vi "Main.vi"() -> ()   [LabVIEW 2020] (continued)
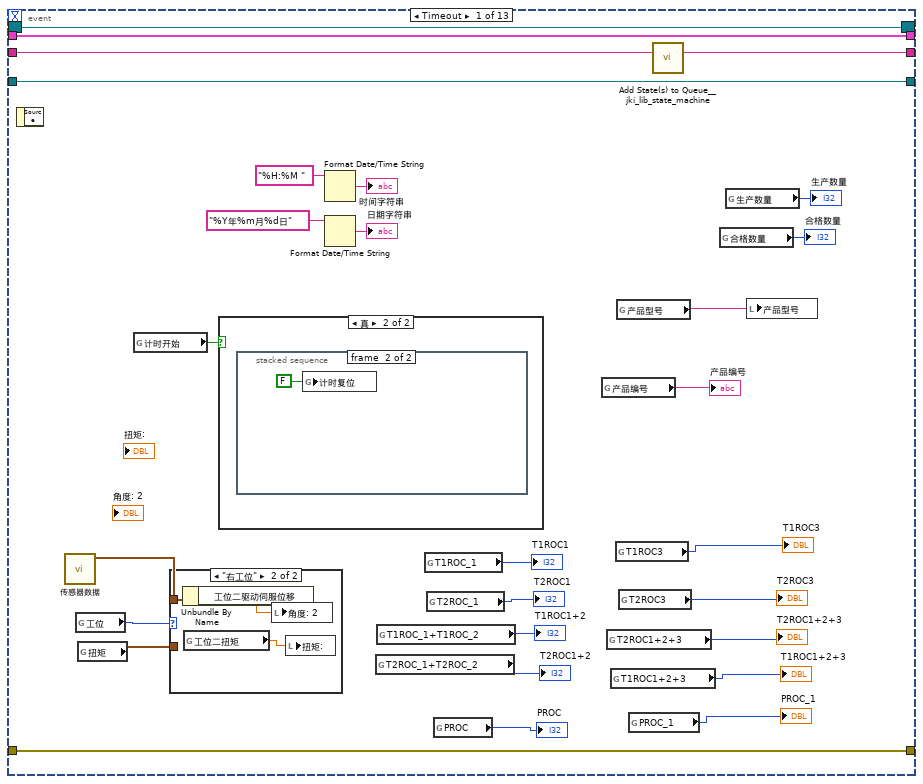
[diagram p2: hidden frame]
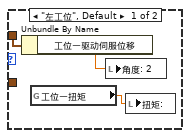
[diagram p3: hidden frame]
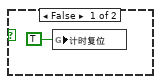
[diagram p4: hidden frame]
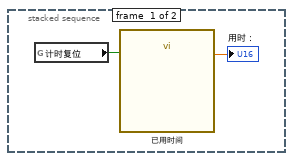
[diagram p5: hidden frame]
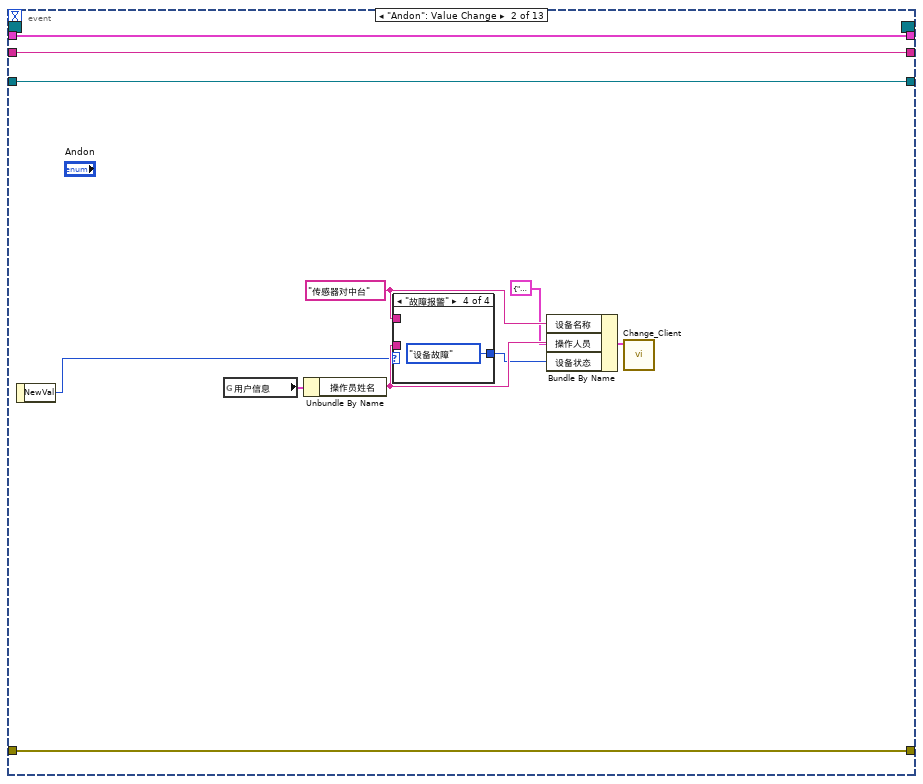
[diagram p6: hidden frame]
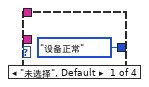
[diagram p7: hidden frame]
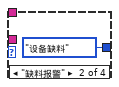
[diagram p8: hidden frame]
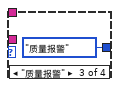
[diagram p9: hidden frame]
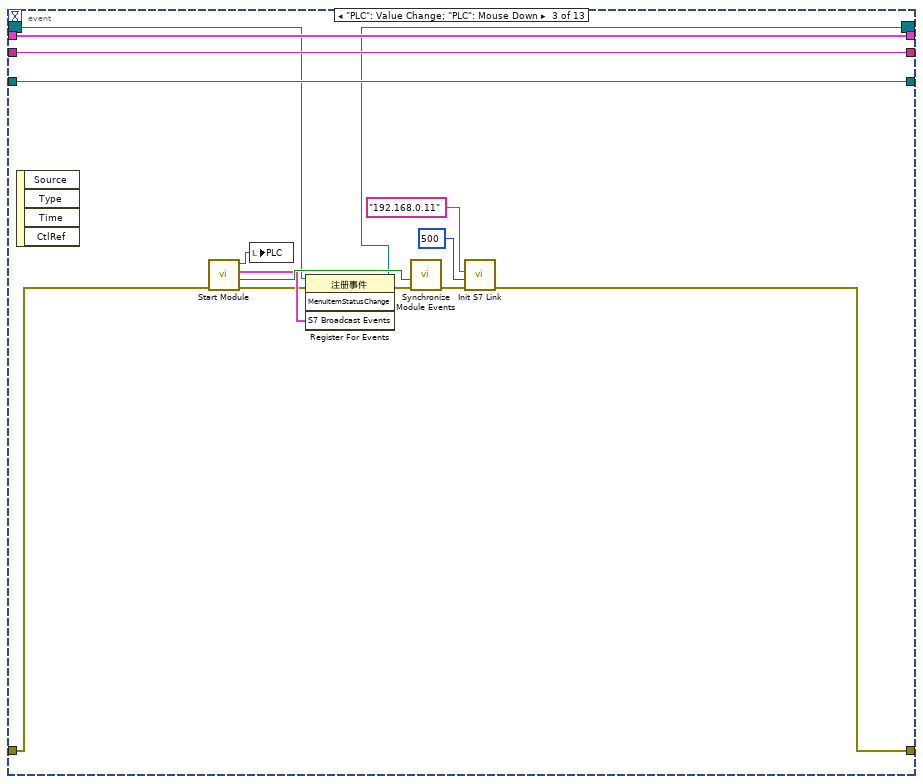
[diagram p10: hidden frame]
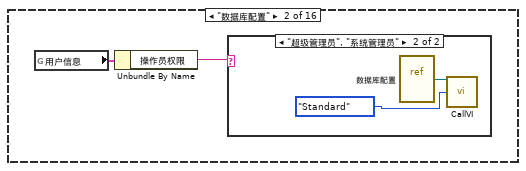
[diagram p12: hidden frame]
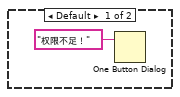
[diagram p13: hidden frame]
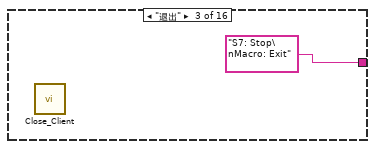
[diagram p14: hidden frame]
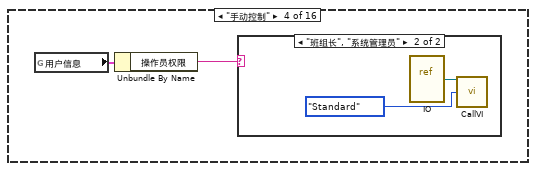
[diagram p15: hidden frame]
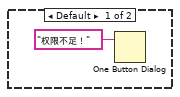
[diagram p16: hidden frame]
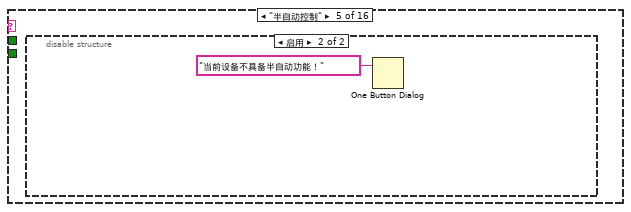
[diagram p17: hidden frame]
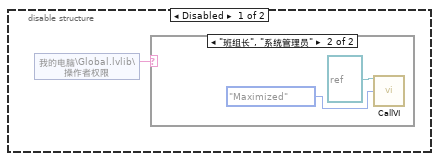
[diagram p18: hidden frame]
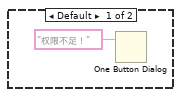
[diagram p19: hidden frame]
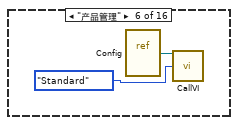
[diagram p20: hidden frame]
            }
            n123 = call <vilib>:"Add State(s) to Queue__jki_lib_state_machine.vi"("State(s) in (\"\")"=w114, "State(s) at Back (\"\")"=w107) -> ("States Out"=w112:string)  [unwired: 13 in]
          }
          event User Event {
            n124 = event-data() -> ("Init?"=w181:bool)  [unwired: 1 in, 1 out]
            n125 = local write "PLC"(w181) -> ()
            n126 = call <vilib>:"Add State(s) to Queue__jki_lib_state_machine.vi"("State(s) in (\"\")"=w176) -> ("States Out"=w177:string)  [unwired: 14 in]
          }
          event User Event {
            n127 = event-data() -> ("Running?"=w188:bool)  [unwired: 1 in]
            n128 = local write "PLC"(w188) -> ()
            n129 = call <vilib>:"Add State(s) to Queue__jki_lib_state_machine.vi"("State(s) in (\"\")"=w183) -> ("States Out"=w184:string)  [unwired: 14 in]
          }
          event User Event {
            n130 = event-data() -> ()  [unwired: 1 in, 7 out]
            n131 = local write "PLC"(FALSE ("PLC")) -> ()
            n132 = call <vilib>:"Add State(s) to Queue__jki_lib_state_machine.vi"("State(s) in (\"\")"=w192) -> ("States Out"=w193:string)  [unwired: 14 in]
          }
          event User Event {
            n133 = event-data() -> ("Error"=w204:errorcluster)  [unwired: 1 in]
            n134 = Merge Errors(w204, w203) -> (w202:errorcluster)
            n135 = disable-structure shown="禁用" {
              disable-tunnel: ["S7: Stop\nS7: Initialize\nIdle" _] -> w197
              frame Disabled {
              }
              frame Enabled {
              }
            }
            n136 = call <vilib>:"Add State(s) to Queue__jki_lib_state_machine.vi"("State(s) in Front (\"\")"=w197, "State(s) in (\"\")"=w199) -> ("States Out"=w200:string)  [unwired: 13 in]
          }
          event "自动": Mouse Down {
            n137 = event-data() -> ()  [unwired: 1 in, 1 out]
            n138 = local read "自动"() -> (w206:bool)
            n139 = case shown="假" w206 {
              frame False {
                n140 = global read "Global.vi" "工位"() -> (w213:enum16{"左工位", "右工位"})
                n141 = case shown="\"左工位\", 默认" w213 {
                  frame "左工位", Default {
                    n142 = call "设备状态.vi"("工位"=enum16{"工位一", "工位二"}."工位一") -> ("Status_Read"=w215:i16)  [unwired: 10 in]
                    n143 = case shown="5" w215 {
                      frame 0, Default {
                        n144 = One Button Dialog(message="请复位！" ("消息")) -> ()  [unwired: 1 in, 1 out]
                        n145 = call "设备状态.vi"("枚举"=enum16{"Read", "Write"}."Write", "工位"=enum16{"工位一", "工位二"}."工位一", "Status_Write"=i16 0) -> ()  [unwired: 8 in, 1 out]
                      }
                      frame 5 {
                        n146 = vi-ref "Auto.vi"() -> (w222:refnum<vi>)
                        n147 = invoke class="VI" method="Ctrl Val.Set"(reference=w222, "Control Name"="STEP" ("控件名"), "Value"="进入自动" ("控件名")) -> ()  [unwired: 2 in, 5 out]
                      }
                    }
                  }
                  frame "右工位" {
                    n148 = call "设备状态.vi"("工位"=enum16{"工位一", "工位二"}."工位二") -> ("Status_Read"=w224:i16)  [unwired: 10 in]
                    n149 = case shown="5" w224 {
                      frame 0, Default {
                        n150 = One Button Dialog(message="请复位！" ("消息")) -> ()  [unwired: 1 in, 1 out]
                        n151 = call "设备状态.vi"("枚举"=enum16{"Read", "Write"}."Write", "工位"=enum16{"工位一", "工位二"}."工位二", "Status_Write"=i16 0) -> ()  [unwired: 8 in, 1 out]
                      }
                      frame 5 {
                        n152 = vi-ref "Auto2.vi"() -> (w231:refnum<vi>)
                        n153 = invoke class="VI" method="Ctrl Val.Set"(reference=w231, "Control Name"="STEP" ("控件名"), "Value"="进入自动" ("控件名")) -> ()  [unwired: 2 in, 5 out]
                      }
                    }
                  }
                }
              }
              frame True {
                n154 = global read "Global.vi" "工位"() -> (w232:enum16{"左工位", "右工位"})
                n155 = case shown="\"左工位\", 默认" w232 {
                  frame "左工位", Default {
                    n156 = Two Button Dialog(message="确定要退出自动？" ("消息")) -> (T button?=w233:bool)  [unwired: 2 in]
                    n157 = case shown="真" w233 {
                      frame False {
                      }
                      frame True {
                        n158 = vi-ref "Auto.vi"() -> (w237:refnum<vi>)
                        n159 = invoke class="VI" method="Ctrl Val.Set"(reference=w237, "Control Name"="STEP" ("控件名"), "Value"="退出自动" ("控件名")) -> ()  [unwired: 2 in, 5 out]
                      }
                    }
                  }
                  frame "右工位" {
                    n160 = Two Button Dialog(message="确定要退出自动？" ("消息")) -> ()  [unwired: 2 in, 1 out]
                    n161 = vi-ref "Auto2.vi"() -> (w240:refnum<vi>)
                    n162 = invoke class="VI" method="Ctrl Val.Set"(reference=w240, "Control Name"="STEP" ("控件名"), "Value"="退出自动" ("控件名")) -> ()  [unwired: 2 in, 5 out]
                  }
                }
              }
            }
            n163 = call <vilib>:"Add State(s) to Queue__jki_lib_state_machine.vi"("State(s) in (\"\")"=w209) -> ("States Out"=w210:string)  [unwired: 14 in]
          }
          event "布尔": Mouse Down {
            n164 = event-data() -> ()  [unwired: 1 in, 8 out]
            n165 = vi-ref "System.vi"() -> (w249:refnum<vi>)
            n166 = call "CallVI.vi"("VI引用"=w249, "状态"=T4."Standard") -> ()  [unwired: 12 in, 2 out]
            n167 = call <vilib>:"Add State(s) to Queue__jki_lib_state_machine.vi"("State(s) in (\"\")"=w245) -> ("States Out"=w244:string)  [unwired: 14 in]
          }
          event "错误": Mouse Down {
            n168 = event-data() -> ()  [unwired: 1 in, 8 out]
            n169 = vi-ref "报警信息.vi"() -> (w252:refnum<vi>)
            n170 = call "CallVI.vi"("VI引用"=w252, "状态"=T4."Standard") -> ()  [unwired: 12 in, 2 out]
            n171 = call <vilib>:"Add State(s) to Queue__jki_lib_state_machine.vi"("State(s) in (\"\")"=w254) -> ("States Out"=w255:string)  [unwired: 14 in]
          }
          event Panel Close? {
            n172 = event-data() -> ()  [unwired: 1 in, 1 out]
            n173 = global write "Global.vi" "程序关闭"(TRUE ("程序关闭")) -> ()
            n174 = call <vilib>:"Add State(s) to Queue__jki_lib_state_machine.vi"("State(s) in Front (\"\")"="S7: Stop\nMacro: Exit", "State(s) in (\"\")"=w264) -> ("States Out"=w263:string)  [unwired: 13 in]
            n175 = event-data("Discard?"=TRUE) -> ()  [unwired: 1 in, 1 out]
          }
          event "更换产品": Value Change {
            n176 = event-data() -> ("NewVal"=w266:refnum<vi>)  [unwired: 1 in, 5 out]
            n177 = stacked-sequence {
              tunnel: w266 -> [w271]
              frame #0 {
                n178 = stacked-sequence {
                  tunnel: w271 -> [w272]
                  frame #0 {
                    n179 = disable-structure shown="禁用" {
                      disable-tunnel: w272 -> [w274 _]
                      frame Disabled {
                        n180 = call "Call_SubPanal.vi"("VI引用句柄"=w274) -> ("SubPnl引用句柄"=w273:refnum<vi>)  [unwired: 9 in, 1 out]
                      }
                      frame Enabled {
                      }
                    }
                  }
                }
              }
            }
            n181 = call <vilib>:"Add State(s) to Queue__jki_lib_state_machine.vi"("State(s) in (\"\")"=w267) -> ("States Out"=w268:string)  [unwired: 14 in]
          }
        }
      }
      frame "---------- Core ----------" {
        n182 = call <vilib>:"Add State(s) to Queue__jki_lib_state_machine.vi"("State(s) in (\"\")"=w280) -> ("States Out"=w279:string)  [unwired: 14 in]
      }
      frame Default {
        w292 = 42 items=["No error", "Argument error", "Memory is full", "Out of zone", "End of file", "File already open", "Generic file I/O error", "File not found", "File permission error", "Disk is full", "Duplicate path", "Too many files open", "System feature not enabled", "Resource file not found", "Cannot add resource", "Resource not found", "Image not found", "Image memory error", "Pen does not exist", "Config type invalid", "Config token not found", "Config parse error", "Config memory error", "Bad external code format", "Bad external code offset", "External code not present", "Null window", "Destroy window error", "Null menu", "Print aborted", "Bad print record", "Print driver error", "Windows error during printing", "Memory error during printing", "Print dialog error", "Generic print error", "Invalid device refnum", "Device not found", "Device parameter error", "Device unit error", "Cannot open device", "Device call aborted", "Generic error", "Cancelled by user", "Object ID too low", "Object ID too high", "Object not in heap", "Unknown heap", "Unknown object (invalid DefProc)", "Unknown object (DefProc not in table)", "Message out of range", "Invalid (null) method", "Unknown message", "Manager call not supported", "Bad address", "Network operation in progress", "Network operation timed out", "Connection is busy", "Network attribute not supported", "Network error", "Address in use", "System out of memory", "Connection aborted", "Connection refused", "Not connected", "Already connected", "Connection closed", "Initialization error (interapplication manager)", "Bad occurrence", "Wait on unbound occurrence handler", "Occurrence queue overflow", "Datalog type conflict", "Unused", "Unrecognized type (interapplication manager)", "Memory corrupt", "Failed to make temporary DLL", "Old CIN version", "Drag socket not found", "Failed to load drop-object", "Failed to register OLE object", "Failed to release OLE object", "Format specifier type mismatch", "Unknown format specifier", "Too few format specifiers", "Too many format specifiers", "Scan failed", "Newer CIN version", "Error converting to variant", "Runtime menu error", "Password tampered", "Variant attribute not found", "Incompatible variant data type", "Event data is not available", "Event Store is not present", "Occurrence is not found", "Event Queue is not created", "Event info is not available", "Refnum passed is NULL", "Error retrieving Class GUID", "Error retrieving CoClass GUID", "Error retrieving TypeLib GUID.", "Bad built application magic bytes.", "Specific driver is different from the specific driver associated with the Logical Name.", "There is no session opened to the class driver.", "Max Error", "MAX - Error with config objects", "MAX - Error loading configuration", "MAX - Group not supported"]
        # "Current State"
        n183 = Format Into String(format string="Software Exception: Unhandled State \"%s\"." ("message"), error in=w288, w283) -> (resulting string=w291:string, error out=w290:errorcluster)  [unwired: 1 in]
        n184 = call <vilib>:"Error Cluster From Error Code.vi"("show call chain? (False)"=TRUE, "error in (no error)"=w290, "error message (\"\")"=w291, "error code (0)"=w292) -> ("error out"=w289:errorcluster)  [unwired: 5 in]
        n185 = call <vilib>:"Add State(s) to Queue__jki_lib_state_machine.vi"("State(s) in (\"\")"=w287) -> ("States Out"=w286:string)  [unwired: 14 in]
      }
      frame "Initialize Core Data" {
        # "originally closed?"
        # "exe?"
        n186 = property class="VI"() -> ("Front Panel.Open"=w303:bool)  [unwired: 2 in, 2 out]
        n187 = property class="App"() -> ("App.Kind"=w302:T5)  [unwired: 2 in, 2 out]
        n188 = control-ref of="Current VI Reference"() -> (w296:refnum<vi>)
        n189 = Not(x=w303) -> (.not. x?=w300:bool)
        n190 = Equal?(x=w302, y=T5."Run Time System" ("Application:Kind")) -> (x = y?=w299:bool)
        n191 = Or(x=w300, y=w299) -> (x .or. y?=w297:bool)
        n192 = Bundle By Name(cluster=w298, "Core.Current VI Reference"=w296, "Core.Close Panel on Exit?"=w297) -> (w305:T8)
        n193 = call <vilib>:"Add State(s) to Queue__jki_lib_state_machine.vi"("State(s) in (\"\")"=w307) -> ("States Out"=w306:string)  [unwired: 14 in]
      }
      frame "Error Handler" {
        n194 = call <vilib>:"General Error Handler.vi"("error in (no error)"=w311) -> ()  [unwired: 10 in, 5 out]
        n195 = call <vilib>:"Add State(s) to Queue__jki_lib_state_machine.vi"("State(s) in Front (\"\")"="/* Post Error States", "State(s) in (\"\")"=w315) -> ("States Out"=w314:string)  [unwired: 13 in]
      }
      frame "Exit" {
        n196 = call <vilib>:"Add State(s) to Queue__jki_lib_state_machine.vi"("State(s) in (\"\")"=w322) -> ("States Out"=w321:string)  [unwired: 14 in]
      }
      frame "--------- Library --------" {
        n197 = call <vilib>:"Add State(s) to Queue__jki_lib_state_machine.vi"("State(s) in (\"\")"=w328) -> ("States Out"=w327:string)  [unwired: 14 in]
      }
      frame "S7: Initialize" {
        n198 = property on="PLC" class="Bool (严格)"("Val(Sgnl)"=FALSE ("值(信号)")) -> ()  [unwired: 2 in, 2 out]
      }
      frame "S7: Stop" {
        n199 = call "Stop Module.vi"("error in (no error)"=w337) -> ("error out"=w336:errorcluster)  [unwired: 10 in]
        n200 = call <vilib>:"Add State(s) to Queue__jki_lib_state_machine.vi"("State(s) in (\"\")"=w338) -> ("States Out"=w339:string)  [unwired: 14 in]
      }
      frame "---------- Data ----------" {
        n201 = call <vilib>:"Add State(s) to Queue__jki_lib_state_machine.vi"("State(s) in (\"\")"=w347) -> ("States Out"=w346:string)  [unwired: 14 in]
      }
      frame "Data: Initialize" {
        w353 = T9 {"Current VI Reference"=refnum, "Close Panel on Exit?"=FALSE}  # Core
        w355 = TRUE  # Your Boolean data
        w354 = ""  # Your string data
        n202 = vi-ref "扭矩.vi"() -> (w349:refnum<vi>)
        n203 = call "CallVI.vi"("VI引用"=w349, "状态"=T4."Hidden") -> ()  [unwired: 12 in, 2 out]
        n204 = global write "Global.vi" "计时开始"(FALSE ("计时结束")) -> ()
        n205 = Bundle("Core"=w353, "Your Boolean data"=w355, "Your string data"=w354) -> (w357:T8)  [unwired: 1 in]
        n206 = call <vilib>:"Add State(s) to Queue__jki_lib_state_machine.vi"("State(s) in (\"\")"=w359) -> ("States Out"=w358:string)  [unwired: 14 in]
      }
      frame "Data: Cleanup" {
        n207 = Unbundle By Name(w362) -> ("Core.Current VI Reference"=w365:refnum<vi>)
        n208 = Close Reference(reference=w365, error in (no error)=w364) -> (error out=w363:errorcluster)
        n209 = call <vilib>:"Add State(s) to Queue__jki_lib_state_machine.vi"("State(s) in (\"\")"=w367) -> ("States Out"=w366:string)  [unwired: 14 in]
      }
      frame "---------- UI ----------" {
        # "Do not put any code in this frame.\n(It is a separator no-op. You can make a copy of this frame to create a new UI frame)"
        n210 = call <vilib>:"Add State(s) to Queue__jki_lib_state_machine.vi"("State(s) in (\"\")"=w373) -> ("States Out"=w372:string)  [unwired: 14 in]
      }
      frame "UI: Initialize" {
        n211 = global read "Global.vi" "工位"() -> (w374:enum16{"左工位", "右工位"})
        n212 = disable-structure shown="禁用" {
          frame Disabled {
            n213 = vi-ref "Auto2.vi"() -> (w396:refnum<vi>)
            n214 = property class="VI"(reference=w396) -> (reference out=w397:refnum<vi>, "FP.State"=w398:T4)  [unwired: 1 in, 1 out]
            n215 = case shown="\"Invalid\", \"Closed\"" w398 {
              tunnel: _ -> [w404 w406]
              tunnel: w397 -> [w405 w407]
              tunnel: [w403 w407] -> w399
              tunnel: [w402 w406] -> w400
              frame "Standard", Default {
                n216 = invoke class="VI" method="FP.Close"(reference=w405, error in=w404) -> (reference out=w403:refnum<vi>, error out=w402:errorcluster)  [unwired: 1 in, 1 out]
              }
              frame "Invalid", "Closed" {
              }
            }
            n217 = invoke class="SubPnl" method="Insert VI"(error in=w400, "VI Ref"=w399) -> (reference=w393:refnum<vi>, error out=w401:errorcluster)  [unwired: 1 in, 3 out]
            n218 = invoke class="VI" method="Run VI"(reference=w399, error in=w401, "Wait until done"=FALSE ("结束前等待"), "Auto Dispose Ref"=TRUE ("自动销毁引用")) -> ()  [unwired: 1 in, 5 out]
          }
          frame Enabled {
          }
        }
        n219 = case shown="\"右工位\"" w374 {
          tunnel: [w391 w392] -> w382
          frame "左工位", Default {
            n220 = vi-ref "Auto.vi"() -> (w391:refnum<vi>)
          }
          frame "右工位" {
            n221 = vi-ref "Auto2.vi"() -> (w392:refnum<vi>)
          }
        }
        n222 = control-ref of="工位一子面板"() -> (w376:refnum<vi>)
        n223 = property class="VI"(reference=w382) -> (reference out=w381:refnum<vi>, "FP.State"=w380:T4)  [unwired: 1 in, 1 out]
        n224 = case shown="\"Invalid\", \"Closed\"" w380 {
          tunnel: w385 -> [w410 w412]
          tunnel: w381 -> [w411 w413]
          tunnel: [w409 w413] -> w379
          tunnel: [w408 w412] -> w378
          frame "Standard", Default {
            n225 = invoke class="VI" method="FP.Close"(reference=w411, error in=w410) -> (reference out=w409:refnum<vi>, error out=w408:errorcluster)  [unwired: 1 in, 1 out]
          }
          frame "Invalid", "Closed" {
          }
        }
        n226 = invoke class="SubPnl" method="Insert VI"(reference=w376, error in=w378, "VI Ref"=w379) -> (error out=w377:errorcluster)  [unwired: 1 in, 3 out]
        n227 = invoke class="VI" method="Run VI"(reference=w379, error in=w377, "Wait until done"=FALSE ("结束前等待"), "Auto Dispose Ref"=TRUE ("自动销毁引用")) -> (error out=w375:errorcluster)  [unwired: 1 in, 4 out]
        n228 = call <vilib>:"Add State(s) to Queue__jki_lib_state_machine.vi"("State(s) in (\"\")"=w390) -> ("States Out"=w389:string)  [unwired: 14 in]
      }
      frame "UI: Init" {
        n229 = stacked-sequence {
          tunnel: w415 -> [_ _ _ _ _]
          frame #0 {
            n230 = global read "Global.vi" "工位"() -> (→"工位":enum16{"左工位", "右工位"})
            n231 = global write "Global.vi" "程序关闭"(FALSE ("程序关闭")) -> ()
            n232 = control-ref of="动态标定"() -> (w422:refnum<vi>)
            n233 = control-ref of="传感器特性"() -> (w425:refnum<vi>)
            n234 = control-ref of="程序固化"() -> (w424:refnum<vi>)
            n235 = control-ref of="静态标定"() -> (w423:refnum<vi>)
            n236 = control-ref of="可信度"() -> (w421:refnum<vi>)
            n237 = global write "Global.vi" "动态优化引用句柄"(w422) -> ()
            n238 = global write "Global.vi" "传感器特性用句柄"(w425) -> ()
            n239 = global write "Global.vi" "可信度检测引用句柄"(w421) -> ()
            n240 = global write "Global.vi" "程序固化引用句柄"(w424) -> ()
            n241 = global write "Global.vi" "静态标定引用句柄"(w423) -> ()
          }
          frame #1 {
            w432 = 0
            n242 = shared-variable "我的电脑\\Global.lvlib\\工位追溯码"("   " ("工位追溯码")) -> ()  [unwired: 1 in, 1 out]
            n243 = global write "Global.vi" "生产数量"(w432) -> ()
            n244 = global write "Global.vi" "合格数量"(w432) -> ()
            n245 = global read "用户信息.vi" "用户信息"() -> (w430:T7)
            n246 = Unbundle By Name(w430) -> ("联机模式"=w427:enum16{"单机", "追溯"}, "操作员姓名"=→"userName":string, "操作员权限"=→"userStatus":string)
            n247 = case shown="\"追溯\"" w427 {
              tunnel: ["联网" ("connectionMode") "单机" ("connectionMode")] -> w433
              frame "追溯" {
              }
              frame "单机", Default {
              }
            }
            "connectionMode" <- w433
          }
          frame #2 {
            n248 = control-ref of="提示信息"() -> (w437:refnum<vi>)
            n249 = control-ref of="自动"() -> (w438:refnum<vi>)
            n250 = control-ref of="错误"() -> (w439:refnum<vi>)
            n251 = control-ref of="Result"() -> (w440:refnum<vi>)
            n252 = control-ref of="更换产品"() -> (w436:refnum<vi>)
            n253 = global write "Global.vi" "提示信息"(w437) -> ()
            n254 = global write "Global.vi" "程序自动"(w438) -> ()
            n255 = global write "Global.vi" "报警图标"(w439) -> ()
            n256 = global write "Global.vi" "Result"(w440) -> ()
            n257 = global write "Global.vi" "更换产品"(w436) -> ()
          }
          frame #3 {
            n258 = global read "Global.vi" "Result"() -> (w443:refnum<vi>)
            n259 = property class="Tbl"(reference=w443, "Row Headers[]"=string[] [], "Value"=string[][] []) -> ()  [unwired: 1 in, 2 out]
          }
          frame #4 {
            n260 = call "Start_Client.vi"() -> ()  [unwired: 12 in]
          }
        }
        n261 = call <vilib>:"Add State(s) to Queue__jki_lib_state_machine.vi"("State(s) in (\"\")"=w419) -> ("States Out"=w418:string)  [unwired: 14 in]
      }
      frame "UI: Config" {
        n262 = vi-ref "Config.vi"() -> (w445:refnum<vi>)
        n263 = call "CallVI.vi"("VI引用"=w445, "状态"=T4."Standard") -> ()  [unwired: 12 in, 2 out]
        n264 = call <vilib>:"Add State(s) to Queue__jki_lib_state_machine.vi"("State(s) in (\"\")"=w451) -> ("States Out"=w450:string)  [unwired: 14 in]
      }
      frame "UI: Cursor Set" {
        # "Argument"
        n265 = case shown="\"Idle\", 默认" w454 {
          tunnel: w456 -> [w461 w463]
          tunnel: [w460 w462] -> w455
          frame "Idle", Default {
            n266 = call <vilib>:"Unset Busy.vi"("error in (no error)"=w461) -> ("error out"=w460:errorcluster)  [unwired: 10 in]
          }
          frame "Busy" {
            n267 = call <vilib>:"Set Busy.vi"("error in (no error)"=w463) -> ("error out"=w462:errorcluster)  [unwired: 9 in, 1 out]
          }
        }
        n268 = call <vilib>:"Add State(s) to Queue__jki_lib_state_machine.vi"("State(s) in (\"\")"=w459) -> ("States Out"=w458:string)  [unwired: 14 in]
      }
      frame "UI: Front Panel State" {
        # "Argument"
        n269 = Unbundle By Name(w468) -> ("Core.Current VI Reference"=w467:refnum<vi>)
        n270 = case shown="\"Close\"" w466 {
          tunnel: w470 -> [w476 w489]
          tunnel: [w478 w490] -> w469
          tunnel: w467 -> [w477 w487]
          frame "Open", Default {
            n271 = property class="VI"(reference=w477, error in=w476) -> (reference out=w474:refnum<vi>, error out=w475:errorcluster, "Front Panel.Open"=w473:bool)
            n272 = case shown="假" w473 {
              tunnel: [w481 w484] -> w478
              tunnel: w475 -> [w480 w484]
              tunnel: w474 -> [w479 _]
              frame False {
                n273 = invoke class="VI" method="FP.Open"(reference=w479, error in=w480, "Activate"=TRUE, "State"=T4."Standard") -> (error out=w481:errorcluster)  [unwired: 1 in, 4 out]
              }
              frame True {
              }
            }
          }
          frame "Close" {
            n274 = property class="VI"(reference=w487, error in=w489) -> (reference out=w486:refnum<vi>, error out=w488:errorcluster, "Front Panel.Open"=w485:bool)
            n275 = case shown="真" w485 {
              tunnel: [w491 w494] -> w490
              tunnel: w488 -> [w491 w493]
              tunnel: w486 -> [_ w492]
              frame False {
              }
              frame True {
                n276 = invoke class="VI" method="FP.Close"(reference=w492, error in=w493) -> (error out=w494:errorcluster)  [unwired: 1 in, 2 out]
              }
            }
          }
        }
        n277 = call <vilib>:"Add State(s) to Queue__jki_lib_state_machine.vi"("State(s) in (\"\")"=w472) -> ("States Out"=w471:string)  [unwired: 14 in]
      }
      frame "---------- Macro ----------" {
        n278 = call <vilib>:"Add State(s) to Queue__jki_lib_state_machine.vi"("State(s) in (\"\")"=w500) -> ("States Out"=w499:string)  [unwired: 14 in]
      }
      frame "Macro: Initialize" {
        n279 = call <vilib>:"Add State(s) to Queue__jki_lib_state_machine.vi"("State(s) in Front (\"\")"="Data: Initialize\nInitialize Core Data\nS7: Initialize\nIdle\nIdle\nUI: Init\nUI: Front Panel State >> Open\nUI: Initialize\nUI: Config", "State(s) in (\"\")"=w507) -> ("States Out"=w506:string)  [unwired: 13 in]
      }
      frame "Macro: Exit" {
        n280 = Unbundle By Name(w516) -> ("Core.Close Panel on Exit?"=w515:bool)
        n281 = Quit LabVIEW() -> ()  [unwired: 1 in]
        n282 = Select(t="UI: Front Panel State >> Close", s=w515, f="") -> (s? t:f=w512:string)
        n283 = call <vilib>:"Add State(s) to Queue__jki_lib_state_machine.vi"("State(s) in (\"\")"=w512, "State(s) at Back (\"\")"="Data: Cleanup\nExit") -> ("States Out"=w510:string)  [unwired: 13 in]
        n284 = call <vilib>:"Add State(s) to Queue__jki_lib_state_machine.vi"("State(s) in Front (\"\")"=w510, "State(s) in (\"\")"=w519) -> ("States Out"=w518:string)  [unwired: 13 in]
      }
    }
  }
  n285 = call-dynamic "Cleanup.vi"("MenuStrip in"=w6) -> ()  [unwired: 10 in, 1 out]
